vi "project 1.vi"() -> ()   [LabVIEW 2018]
panel:
  out "Your Oder will be prepaded in":dbl
  in  "Pay bill and conform":bool
  out "Discount":string
  out "Total bill":dbl
  out "Price 5":dbl
  in  "Quentity 5":dbl=1.0 min=1.0 max=10.0
  in  "Item Number 5":bool
  out "Price 4":dbl
  in  "Quentity 4":dbl=1.0 min=1.0 max=10.0
  in  "Item Number 4":bool
  out "Price 3":dbl
  in  "Quentity 3":dbl=1.0 min=1.0 max=10.0
  in  "Item Number 3":bool
  out "Price 2":dbl
  in  "Quentity 2":dbl=1.0 min=1.0 max=10.0
  in  "Item Number 2":bool
  out "Price":dbl
  in  "Quentity":dbl=1.0 min=1.0 max=10.0
  in  "Item Number 01":bool
  # "food Odering System"
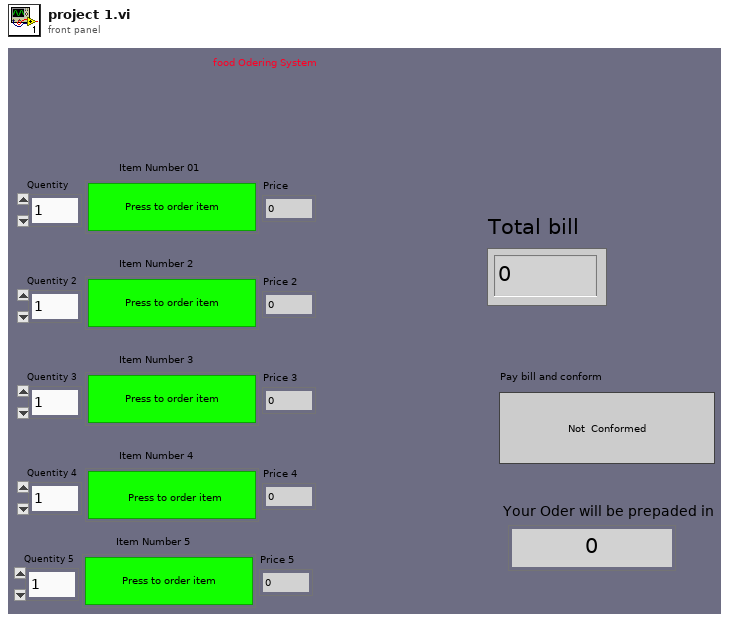
[diagram p1: front panel]
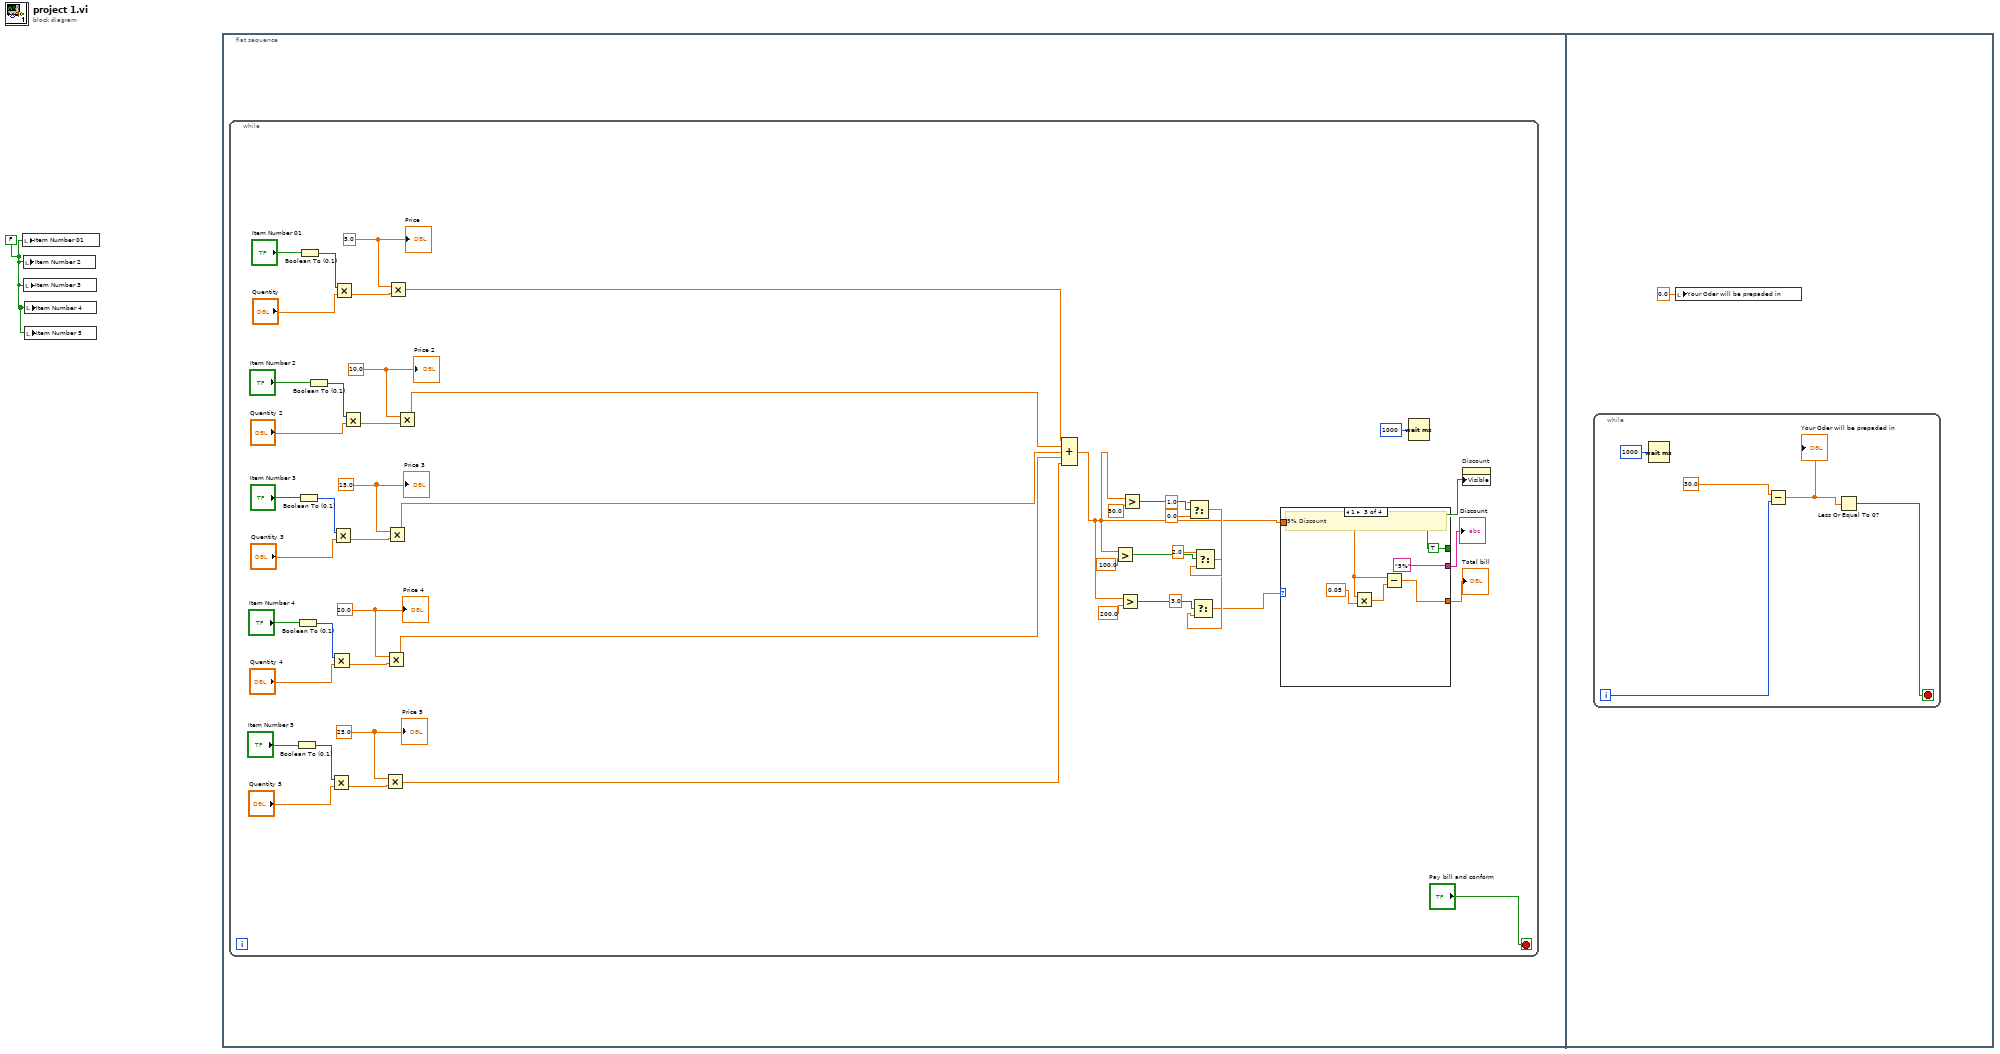
[diagram p0: block diagram]
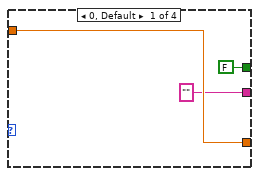
[diagram p2: hidden frame]
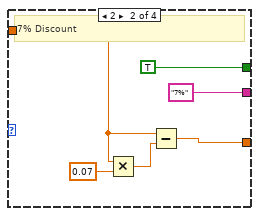
[diagram p3: hidden frame]
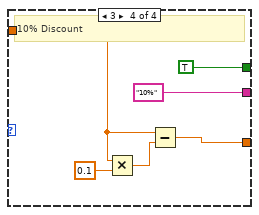
[diagram p4: hidden frame]
diagram:
  w1 = FALSE ("Item Number 01")
  n1 = local write "Item Number 01"(w1) -> ()
  n2 = local write "Item Number 2"(w1) -> ()
  n3 = local write "Item Number 3"(w1) -> ()
  n4 = local write "Item Number 4"(w1) -> ()
  n5 = local write "Item Number 5"(w1) -> ()
  n6 = flat-sequence {
    frame #0 {
      n7 = while {
        stop <- "Pay bill and conform" stop-if-true
        w26 = 25.0 ("Price")
        w31 = 20.0 ("Price")
        w36 = 15.0 ("Price")
        w42 = 10.0 ("Price")
        w46 = 5.0 ("Price")
        n8 = Boolean To (0,1)(Boolean="Item Number 5") -> (0, 1=w28:i16)
        n9 = Boolean To (0,1)(Boolean="Item Number 4") -> (0, 1=w33:i16)
        n10 = Boolean To (0,1)(Boolean="Item Number 3") -> (0, 1=w38:i16)
        n11 = Boolean To (0,1)(Boolean="Item Number 01") -> (0, 1=w48:i16)
        n12 = Boolean To (0,1)(Boolean="Item Number 2") -> (0, 1=w41:i16)
        n13 = Multiply(x=w28, y="Quentity 5") -> (x*y=w27:dbl)
        n14 = Multiply(x=w33, y="Quentity 4") -> (x*y=w32:dbl)
        n15 = Multiply(x=w38, y="Quentity 3") -> (x*y=w37:dbl)
        n16 = Multiply(x=w48, y="Quentity") -> (x*y=w47:dbl)
        n17 = Multiply(x=w41, y="Quentity 2") -> (x*y=w43:dbl)
        n18 = Multiply(x=w26, y=w27) -> (x*y=w21:dbl)
        n19 = Multiply(x=w31, y=w32) -> (x*y=w22:dbl)
        n20 = Multiply(x=w36, y=w37) -> (x*y=w23:dbl)
        n21 = Multiply(x=w46, y=w47) -> (x*y=w25:dbl)
        n22 = Multiply(x=w42, y=w43) -> (x*y=w24:dbl)
        n23 = Compound Arithmetic op=ADD(w25, w24, w23, w22, w21) -> (w7:dbl)
        n24 = Greater?(x=w7, y=100.0) -> (0:w14:bool)
        n25 = Greater?(x=w7, y=200.0) -> (0:w11:bool)
        n26 = Greater?(x=w7, y=50.0) -> (0:w17:bool)
        n27 = Select(t=1.0, s=w17, f=0.0) -> (s? t:f=w12:dbl)
        n28 = Select(t=2.0, s=w14, f=w12) -> (s? t:f=w9:dbl)
        n29 = Select(t=3.0, s=w11, f=w9) -> (s? t:f=w8:dbl)
        n30 = case shown="1" w8 {
          tunnel: w7 -> [w53 w57 w63 w69]
          tunnel: [w53 w56 w62 w68] -> w6
          tunnel: ["" ("Discount") "7%" ("Discount") "5%" ("Discount") "10%" ("Discount")] -> w5
          tunnel: [FALSE ("Visible") TRUE ("Visible") TRUE ("Visible") TRUE ("Visible")] -> w2
          frame 0, Default {
          }
          frame 2 {
            # "7% Discount"
            n31 = Multiply(x=w57, y=0.07) -> (x*y=w58:dbl)
            n32 = Subtract(x=w57, y=w58) -> (x-y=w56:dbl)
          }
          frame 1 {
            # "5% Discount"
            n33 = Multiply(x=w63, y=0.05) -> (x*y=w64:dbl)
            n34 = Subtract(x=w63, y=w64) -> (x-y=w62:dbl)
          }
          frame 3 {
            # "10% Discount"
            n35 = Multiply(x=w69, y=0.1) -> (x*y=w70:dbl)
            n36 = Subtract(x=w69, y=w70) -> (x-y=w68:dbl)
          }
        }
        "Total bill" <- w6
        "Discount" <- w5
        n37 = Wait (ms)(milliseconds to wait=u32 1000) -> ()  [unwired: 1 out]
        n38 = property on="Discount" class="Str"("Visible"=w2) -> ()  [unwired: 2 in, 2 out]
        "Price" <- w46
        "Price 2" <- w42
        "Price 3" <- w36
        "Price 4" <- w31
        "Price 5" <- w26
      }
    }
    frame #1 {
      n39 = while {
        i -> [w77]
        stop <- w74 stop-if-true
        n40 = Wait (ms)(milliseconds to wait=u32 1000) -> ()  [unwired: 1 out]
        n41 = Subtract(x=30.0, y=w77) -> (x-y=w75:dbl)
        "Your Oder will be prepaded in" <- w75
        n42 = Less Or Equal To 0?(x=w75) -> (x <= 0?=w74:bool)
      }
      n43 = local write "Your Oder will be prepaded in"(0.0 ("Your Oder will be prepaded in")) -> ()
    }
  }
